vi "UHR-Fleezers Control (host) - Avogadro v2.vi"() -> ()   [LabVIEW 2014] (continued)
          frame Disabled {
            w2902 = FALSE ("Stop Flow")
            n1843 = local write "Stop Flow"(w2902) -> ()
            n1844 = local write "Sample Channel\nFlow"(w2902) -> ()
            n1845 = Concatenate Strings("stop" ("string"), "\r") -> (w2905:string)
            n1846 = VISA Write(VISA resource name=w2903, write buffer=w2905) -> ()  [unwired: 1 in, 3 out]
          }
          frame Enabled {
          }
        }
      }
      event "Flow rate (uL/h)": Value Change {
        n1847 = event-data() -> ()  [unwired: 7 out]
        n1848 = disable-structure shown="Disabled" {
          disable-tunnel: w2907 -> [w2909 _]
          frame Disabled {
            n1849 = Number To Decimal String(number="Flow rate (uL/h)") -> (decimal integer string=w2913:string)  [unwired: 1 in]
            n1850 = Concatenate Strings("irate  " ("string"), w2913, " u/h" ("string"), "\r") -> (w2912:string)
            n1851 = VISA Write(VISA resource name=w2909, write buffer=w2912) -> ()  [unwired: 1 in, 3 out]
          }
          frame Enabled {
          }
        }
      }
      event "Flush Sample": Value Change {
        n1852 = event-data() -> ()  [unwired: 7 out]
        n1853 = disable-structure shown="Disabled" {
          disable-tunnel: ["Flush Sample" _] -> w2916
          disable-tunnel: w2915 -> [w2922 _]
          frame Disabled {
            n1854 = flat-sequence {
              tunnel: w2922 -> [w2963]
              tunnel: [w2943] -> w2926
              tunnel: [w2939] -> w2925
              tunnel: ["Volume (uL)"] -> w2921
              tunnel: ["Flush rate (uL/m)"] -> w2920
              tunnel: w2926 -> [w2967]
              tunnel: [w2967] -> w2924
              tunnel: w2925 -> [w2966]
              tunnel: w2924 -> [w2972]
              frame #0 {
                # "set paramaters (rate, volume) for flush, clear volume"
                n1855 = Number To Decimal String(number="Flush rate (uL/m)") -> (decimal integer string=w2959:string)  [unwired: 1 in]
                n1856 = Concatenate Strings("irate  " ("string"), w2959, " u/m" ("string"), "\r") -> (w2961:string)
                n1857 = VISA Write(VISA resource name=w2963, write buffer=w2961) -> (VISA resource name out=w2957:refnum<visa-resource-name>)  [unwired: 1 in, 2 out]
                n1858 = Reciprocal(x="Flush rate (uL/m)") -> (1/x=w2942:dbl)
                n1859 = Number To Decimal String(number="Volume (uL)") -> (decimal integer string=w2948:string)  [unwired: 1 in]
                n1860 = Multiply(x="Volume (uL)", y=w2942) -> (x*y=w2941:dbl)
                n1861 = Concatenate Strings("tvolume  " ("string"), w2948, " u" ("string"), "\r") -> (w2946:string)
                n1862 = Multiply(x=w2941, y=60000.0) -> (x*y=w2939:dbl)
                n1863 = VISA Write(VISA resource name=w2957, write buffer=w2946) -> (VISA resource name out=w2945:refnum<visa-resource-name>)  [unwired: 1 in, 2 out]
                n1864 = Concatenate Strings("cvolume" ("string"), "\r") -> (w2944:string)
                n1865 = VISA Write(VISA resource name=w2945, write buffer=w2944) -> (VISA resource name out=w2955:refnum<visa-resource-name>)  [unwired: 1 in, 2 out]
                n1866 = Concatenate Strings("irun" ("string"), "\r") -> (w2953:string)
                n1867 = VISA Write(VISA resource name=w2955, write buffer=w2953) -> (VISA resource name out=w2943:refnum<visa-resource-name>)  [unwired: 1 in, 2 out]
              }
              frame #1 {
                # "Have to wait until\nflow is done to reset\nrate"
                n1868 = Add(x=w2966, y=100.0) -> (x+y=w2965:dbl)
                n1869 = Wait (ms)(milliseconds to wait=w2965) -> ()  [unwired: 1 out]
              }
              frame #2 {
                # "reset flow rate to usual flow rate"
                n1870 = local read "Flow rate (uL/h)"() -> (w2978:dbl)
                n1871 = Number To Decimal String(number=w2978) -> (decimal integer string=w2976:string)  [unwired: 1 in]
                n1872 = Concatenate Strings("irate  " ("string"), w2976, " u/h" ("string"), "\r") -> (w2974:string)
                n1873 = VISA Write(VISA resource name=w2972, write buffer=w2974) -> (VISA resource name out=w2968:refnum<visa-resource-name>)  [unwired: 1 in, 2 out]
                n1874 = Concatenate Strings("cvolume" ("string"), "\r") -> (w2969:string)
                n1875 = VISA Write(VISA resource name=w2968, write buffer=w2969) -> ()  [unwired: 1 in, 3 out]
              }
            }
            n1876 = local read "Save Event Log?"() -> (w2918:bool)
            n1877 = local read "Saving..."() -> (w2917:bool)
            n1878 = And(x=w2918, y=w2917) -> (x .and. y?=w2919:bool)
            n1879 = case shown="True" w2919 {
              tunnel: w2921 -> [_ w2928]
              tunnel: w2920 -> [_ w2927]
              frame False {
              }
              frame True {
                n1880 = Number To Decimal String(number=w2928) -> (decimal integer string=w2932:string)  [unwired: 1 in]
                n1881 = Number To Decimal String(number=w2927) -> (decimal integer string=w2934:string)  [unwired: 1 in]
                n1882 = local read "log file ref"() -> (w2929:refnum<file>)
                n1883 = local read "Time (s)"() -> (w2930:dbl)
                n1884 = Concatenate Strings("pump 2 flushing ", w2932, " uL at ", w2934, " ul/min") -> (w2936:string)
                n1885 = call "write to event log.vi"("log file ref"=w2929, "time"=w2930, "input string"=w2936) -> ()  [unwired: 8 in]
              }
            }
          }
          frame Enabled {
          }
        }
      }
      event "Flush Pump 3": Value Change {
        n1886 = event-data() -> ()  [unwired: 7 out]
        n1887 = disable-structure shown="Disabled" {
          disable-tunnel: ["Flush Pump 3" _] -> w2980
          disable-tunnel: w2979 -> [w2986 _]
          frame Disabled {
            n1888 = flat-sequence {
              tunnel: w2986 -> [w3001]
              tunnel: ["Flush rate (uL/m) P3"] -> w2982
              tunnel: ["Volume (uL) P3"] -> w2981
              frame #0 {
                # "set paramaters (rate, volume) for flush, clear volume"
                n1889 = Number To Decimal String(number="Flush rate (uL/m) P3") -> (decimal integer string=w3021:string)  [unwired: 1 in]
                n1890 = local write "Inject Pump 3"(TRUE ("Inject Pump 3")) -> ()
                n1891 = Concatenate Strings("irate  " ("string"), w3021, " u/m" ("string"), "\r") -> (w3023:string)
                n1892 = VISA Write(VISA resource name=w3001, write buffer=w3023) -> (VISA resource name out=w3019:refnum<visa-resource-name>)  [unwired: 1 in, 2 out]
                n1893 = Reciprocal(x="Flush rate (uL/m) P3") -> (1/x=w3005:dbl)
                n1894 = Number To Decimal String(number="Volume (uL) P3") -> (decimal integer string=w3010:string)  [unwired: 1 in]
                n1895 = Multiply(x="Volume (uL) P3", y=w3005) -> (x*y=w3004:dbl)
                n1896 = Concatenate Strings("tvolume  " ("string"), w3010, " u" ("string"), "\r") -> (w3008:string)
                n1897 = Multiply(x=w3004, y=60.0) -> (x*y=→"HP3 Flush Time (s)":dbl)
                n1898 = VISA Write(VISA resource name=w3019, write buffer=w3008) -> (VISA resource name out=w3007:refnum<visa-resource-name>)  [unwired: 1 in, 2 out]
                n1899 = Concatenate Strings("cvolume" ("string"), "\r") -> (w3006:string)
                n1900 = VISA Write(VISA resource name=w3007, write buffer=w3006) -> (VISA resource name out=w3017:refnum<visa-resource-name>)  [unwired: 1 in, 2 out]
                n1901 = Concatenate Strings("irun" ("string"), "\r") -> (w3015:string)
                n1902 = VISA Write(VISA resource name=w3017, write buffer=w3015) -> ()  [unwired: 1 in, 3 out]
              }
              frame #1 {
                "Flushing P3" <- TRUE ("Flushing P3")
              }
            }
            n1903 = local read "Save Event Log?"() -> (w2984:bool)
            n1904 = local read "Saving..."() -> (w2985:bool)
            n1905 = And(x=w2984, y=w2985) -> (x .and. y?=w2983:bool)
            n1906 = case shown="True" w2983 {
              tunnel: w2982 -> [_ w2989]
              tunnel: w2981 -> [_ w2988]
              frame False {
              }
              frame True {
                n1907 = Number To Decimal String(number=w2988) -> (decimal integer string=w2993:string)  [unwired: 1 in]
                n1908 = Number To Decimal String(number=w2989) -> (decimal integer string=w2995:string)  [unwired: 1 in]
                n1909 = local read "log file ref"() -> (w2990:refnum<file>)
                n1910 = local read "Time (s)"() -> (w2991:dbl)
                n1911 = Concatenate Strings("pump 3 flushing ", w2993, " uL at ", w2995, " ul/min") -> (w2997:string)
                n1912 = call "write to event log.vi"("log file ref"=w2990, "time"=w2991, "input string"=w2997) -> ()  [unwired: 8 in]
              }
            }
          }
          frame Enabled {
          }
        }
      }
      event "Flush Pump 1": Value Change {
        n1913 = event-data() -> ()  [unwired: 7 out]
        n1914 = disable-structure shown="Disabled" {
          disable-tunnel: ["Flush Pump 1" _] -> w3027
          disable-tunnel: w3026 -> [w3033 _]
          frame Disabled {
            n1915 = flat-sequence {
              tunnel: [w3054] -> w3035
              tunnel: w3033 -> [w3049]
              tunnel: ["Volume (uL) P1"] -> w3029
              tunnel: ["Flush rate (uL/m) P1"] -> w3028
              tunnel: w3035 -> [_]
              frame #0 {
                # "set paramaters (rate, volume) for flush, clear volume"
                n1916 = local write "Inject Pump 1"(TRUE ("Inject Pump 1")) -> ()
                n1917 = Number To Decimal String(number="Flush rate (uL/m) P1") -> (decimal integer string=w3070:string)  [unwired: 1 in]
                n1918 = Concatenate Strings("irate  " ("string"), w3070, " u/m" ("string"), "\r") -> (w3072:string)
                n1919 = VISA Write(VISA resource name=w3049, write buffer=w3072) -> (VISA resource name out=w3068:refnum<visa-resource-name>)  [unwired: 1 in, 2 out]
                n1920 = Reciprocal(x="Flush rate (uL/m) P1") -> (1/x=w3053:dbl)
                n1921 = Number To Decimal String(number="Volume (uL) P1") -> (decimal integer string=w3059:string)  [unwired: 1 in]
                n1922 = Multiply(x="Volume (uL) P1", y=w3053) -> (x*y=w3052:dbl)
                n1923 = Concatenate Strings("tvolume  " ("string"), w3059, " u" ("string"), "\r") -> (w3057:string)
                n1924 = Multiply(x=w3052, y=60.0) -> (x*y=→"HP1 Flush Time (s)":dbl)
                n1925 = VISA Write(VISA resource name=w3068, write buffer=w3057) -> (VISA resource name out=w3056:refnum<visa-resource-name>)  [unwired: 1 in, 2 out]
                n1926 = Concatenate Strings("cvolume" ("string"), "\r") -> (w3055:string)
                n1927 = VISA Write(VISA resource name=w3056, write buffer=w3055) -> (VISA resource name out=w3066:refnum<visa-resource-name>)  [unwired: 1 in, 2 out]
                n1928 = Concatenate Strings("irun" ("string"), "\r") -> (w3064:string)
                n1929 = VISA Write(VISA resource name=w3066, write buffer=w3064) -> (VISA resource name out=w3054:refnum<visa-resource-name>)  [unwired: 1 in, 2 out]
              }
              frame #1 {
                "Flushing P1" <- TRUE ("Flushing P3")
              }
            }
            n1930 = local read "Saving..."() -> (w3030:bool)
            n1931 = local read "Save Event Log?"() -> (w3031:bool)
            n1932 = And(x=w3031, y=w3030) -> (x .and. y?=w3032:bool)
            n1933 = case shown="True" w3032 {
              tunnel: w3029 -> [_ w3038]
              tunnel: w3028 -> [_ w3037]
              frame False {
              }
              frame True {
                n1934 = Number To Decimal String(number=w3038) -> (decimal integer string=w3042:string)  [unwired: 1 in]
                n1935 = Number To Decimal String(number=w3037) -> (decimal integer string=w3040:string)  [unwired: 1 in]
                n1936 = local read "log file ref"() -> (w3044:refnum<file>)
                n1937 = local read "Time (s)"() -> (w3045:dbl)
                n1938 = Concatenate Strings("pump 1 flushing ", w3042, " uL at ", w3040, " ul/min") -> (w3036:string)
                n1939 = call "write to event log.vi"("log file ref"=w3044, "time"=w3045, "input string"=w3036) -> ()  [unwired: 8 in]
              }
            }
          }
          frame Enabled {
          }
        }
      }
      event "Clear Volume": Value Change {
        n1940 = event-data() -> ()  [unwired: 7 out]
        n1941 = disable-structure shown="Disabled" {
          disable-tunnel: ["Clear Volume" _] -> w3076
          disable-tunnel: w3075 -> [w3077 _]
          frame Disabled {
            n1942 = Concatenate Strings("cvolume" ("string"), "\r") -> (w3078:string)
            n1943 = VISA Write(VISA resource name=w3077, write buffer=w3078) -> ()  [unwired: 1 in, 3 out]
          }
          frame Enabled {
          }
        }
      }
      event "Clear Volume P3": Value Change {
        n1944 = event-data() -> ()  [unwired: 7 out]
        n1945 = disable-structure shown="Disabled" {
          disable-tunnel: w3082 -> [w3084 _]
          frame Disabled {
            n1946 = Concatenate Strings("cvolume" ("string"), "\r") -> (w3085:string)
            n1947 = VISA Write(VISA resource name=w3084, write buffer=w3085) -> ()  [unwired: 1 in, 3 out]
            n1948 = local write "Clear Volume P3"(FALSE ("Clear Volume P3")) -> ()
          }
          frame Enabled {
          }
        }
      }
      event "Clear Volume P1": Value Change {
        n1949 = event-data() -> ()  [unwired: 7 out]
        n1950 = disable-structure shown="Disabled" {
          disable-tunnel: w3088 -> [w3090 _]
          frame Disabled {
            n1951 = Concatenate Strings("cvolume" ("string"), "\r") -> (w3091:string)
            n1952 = local write "Clear Volume P1"(FALSE ("Clear Volume P1")) -> ()
            n1953 = VISA Write(VISA resource name=w3090, write buffer=w3091) -> ()  [unwired: 1 in, 3 out]
          }
          frame Enabled {
          }
        }
      }
      event "Display On P3": Value Change {
        n1954 = event-data() -> ()  [unwired: 7 out]
        n1955 = disable-structure shown="Disabled" {
          disable-tunnel: w3094 -> [w3095 _]
          frame Disabled {
            n1956 = Select(t="dim 100", s="Display On P3", f="dim 0") -> (s? t:f=w3098:string)
            n1957 = Concatenate Strings(w3098, "\r") -> (w3100:string)
            n1958 = VISA Write(VISA resource name=w3095, write buffer=w3100) -> ()  [unwired: 1 in, 3 out]
          }
          frame Enabled {
          }
        }
      }
      event "Display On P1": Value Change {
        n1959 = event-data() -> ()  [unwired: 7 out]
        n1960 = disable-structure shown="Disabled" {
          disable-tunnel: w3102 -> [w3103 _]
          frame Disabled {
            n1961 = Select(t="dim 100", s="Display On P1", f="dim 0") -> (s? t:f=w3106:string)
            n1962 = Concatenate Strings(w3106, "\r") -> (w3108:string)
            n1963 = VISA Write(VISA resource name=w3103, write buffer=w3108) -> ()  [unwired: 1 in, 3 out]
          }
          frame Enabled {
          }
        }
      }
      event "Retract Pump 3": Value Change {
        n1964 = event-data() -> ()  [unwired: 7 out]
        n1965 = disable-structure shown="Disabled" {
          disable-tunnel: w3110 -> [w3111 _]
          frame Disabled {
            n1966 = local write "Retract Pump 3"(FALSE ("Retract Pump 3")) -> ()
            n1967 = case shown="True" "Retract Pump 3" {
              tunnel: w3111 -> [_ w3114]
              frame False {
              }
              frame True {
                n1968 = Number To Decimal String(number="Retract Rate (uL/m)") -> (decimal integer string=w3132:string)  [unwired: 1 in]
                n1969 = Concatenate Strings("wrate  " ("string"), w3132, " u/m" ("string"), "\r") -> (w3134:string)
                n1970 = VISA Write(VISA resource name=w3114, write buffer=w3134) -> (VISA resource name out=w3125:refnum<visa-resource-name>)  [unwired: 1 in, 2 out]
                n1971 = Number To Decimal String(number="Retract Vol 3 (uL)") -> (decimal integer string=w3127:string)  [unwired: 1 in]
                n1972 = Concatenate Strings("tvolume  " ("string"), w3127, " u" ("string"), "\r") -> (w3124:string)
                n1973 = VISA Write(VISA resource name=w3125, write buffer=w3124) -> (VISA resource name out=w3120:refnum<visa-resource-name>)  [unwired: 1 in, 2 out]
                n1974 = Concatenate Strings("cvolume" ("string"), "\r") -> (w3121:string)
                n1975 = VISA Write(VISA resource name=w3120, write buffer=w3121) -> (VISA resource name out=w3115:refnum<visa-resource-name>)  [unwired: 1 in, 2 out]
                n1976 = Concatenate Strings("wrun" ("string"), "\r") -> (w3116:string)
                n1977 = VISA Write(VISA resource name=w3115, write buffer=w3116) -> ()  [unwired: 1 in, 3 out]
              }
            }
          }
          frame Enabled {
          }
        }
      }
      event "Retract Pump 1": Value Change {
        n1978 = event-data() -> ()  [unwired: 7 out]
        n1979 = disable-structure shown="Disabled" {
          disable-tunnel: w3136 -> [w3137 _]
          frame Disabled {
            n1980 = local write "Retract Pump 1"(FALSE ("Retract Pump 1")) -> ()
            n1981 = case shown="True" "Retract Pump 1" {
              tunnel: w3137 -> [_ w3142]
              frame False {
              }
              frame True {
                n1982 = local read "Retract Rate (uL/m)"() -> (w3140:dbl)
                n1983 = Number To Decimal String(number=w3140) -> (decimal integer string=w3158:string)  [unwired: 1 in]
                n1984 = Concatenate Strings("wrate  " ("string"), w3158, " u/m" ("string"), "\r") -> (w3160:string)
                n1985 = VISA Write(VISA resource name=w3142, write buffer=w3160) -> (VISA resource name out=w3152:refnum<visa-resource-name>)  [unwired: 1 in, 2 out]
                n1986 = Number To Decimal String(number="Retract Vol 1 (uL)") -> (decimal integer string=w3154:string)  [unwired: 1 in]
                n1987 = Concatenate Strings("tvolume  " ("string"), w3154, " u" ("string"), "\r") -> (w3151:string)
                n1988 = VISA Write(VISA resource name=w3152, write buffer=w3151) -> (VISA resource name out=w3148:refnum<visa-resource-name>)  [unwired: 1 in, 2 out]
                n1989 = Concatenate Strings("cvolume" ("string"), "\r") -> (w3149:string)
                n1990 = VISA Write(VISA resource name=w3148, write buffer=w3149) -> (VISA resource name out=w3143:refnum<visa-resource-name>)  [unwired: 1 in, 2 out]
                n1991 = Concatenate Strings("wrun" ("string"), "\r") -> (w3144:string)
                n1992 = VISA Write(VISA resource name=w3143, write buffer=w3144) -> ()  [unwired: 1 in, 3 out]
              }
            }
          }
          frame Enabled {
          }
        }
      }
      event "Flip Green Filter": Value Change {
        n1993 = event-data() -> ()  [unwired: 7 out]
        n1994 = Not(x="Flip Green Filter") -> (.not. x?=w3163:bool)
        n1995 = local write "Flip Green Filter"(w3163) -> ()
        n1996 = flat-sequence {
          tunnel: [w3172] -> w3168
          tunnel: [w3171] -> w3167
          tunnel: w3162 -> [w3170]
          tunnel: [w3175] -> w3166
          tunnel: w3168 -> [w3175]
          tunnel: [w3174] -> w3165
          tunnel: w3167 -> [w3174]
          tunnel: w3166 -> [w3179]
          tunnel: w3165 -> [w3178]
          tunnel: [w3177] -> w3169
          frame #0 {
            n1997 = xnode "Read/Write Control"("FPGA VI Reference In"=w3170, "Green Filter Flipper"=TRUE) -> ("FPGA VI Reference Out"=w3172:T40, "error out"=w3171:errorcluster)  [unwired: 1 in]
          }
          frame #1 {
            n1998 = Wait (ms)(milliseconds to wait=u32 100) -> ()  [unwired: 1 out]
          }
          frame #2 {
            n1999 = xnode "Read/Write Control"("FPGA VI Reference In"=w3179, "error in"=w3178, "Green Filter Flipper"=FALSE) -> ("error out"=w3177:errorcluster)  [unwired: 1 out]
          }
        }
      }
      event "Pump 1 contents", "Pump 3 contents": Value Change {
        n2000 = event-data() -> ()  [unwired: 7 out]
        n2001 = local read "Pump 1 contents"() -> (→"Pump 1 cont disp":string)
        n2002 = local read "Pump 3 contents"() -> (→"Pump 3 cont disp":string)
      }
      event "Reset Trap Pos. FB": Value Change {
        n2003 = event-data() -> ()  [unwired: 7 out]
        n2004 = xnode "Read/Write Control"("FPGA VI Reference In"=w3183, "Trap Pos. FB Reset"="Reset Trap Pos. FB") -> ()  [unwired: 1 in, 2 out]
      }
      event "Rem fb disp offset": Value Change {
        n2005 = event-data() -> ()  [unwired: 7 out]
        n2006 = local write "Rem fb disp offset"(FALSE ("Rem fb disp offset")) -> ()
        n2007 = local read "Mean Trap Positions (nm)"() -> (w3186:T6)
        n2008 = local read "FB Trap Pos Offset"() -> (w3188:dbl)
        n2009 = Unbundle By Name(w3186) -> ("T1 X"=w3185:dbl)
        n2010 = Subtract(x=w3188, y=w3185) -> (x-y=w3187:dbl)
        n2011 = local write "FB Trap Pos Offset"(w3187) -> ()
      }
      event "Threshold (nm)": Value Change {
        n2012 = event-data() -> ()  [unwired: 7 out]
        n2013 = flat-sequence {
          tunnel: [w3193] -> w3191
          tunnel: w3190 -> [w3192]
          tunnel: w3191 -> [w3204]
          frame #0 {
            n2014 = xnode "Read/Write Control"("FPGA VI Reference In"=w3192) -> ("FPGA VI Reference Out"=w3196:T40, "error out"=w3195:errorcluster, "FPGA TTrig Thresh"=w3197:i64)  [unwired: 1 in]
            n2015 = local read "Threshold stored (nm)"() -> (w3203:dbl)
            n2016 = local read "Threshold (nm)"() -> (w3193:dbl)
            n2017 = local read "AOM X Cal (nm/MHz)"() -> (w3201:dbl)
            n2018 = Subtract(x=w3193, y=w3203) -> (x-y=w3202:dbl)
            n2019 = Divide(x=w3202, y=w3201) -> (x/y=w3199:dbl)
            n2020 = call "IR AOM freq to word.vi"("Frequency In (MHz)"=w3199) -> ("Frequency Word Out (double)"=w3200:dbl)
            n2021 = To Quad Integer(1:w3200) -> (0:w3198:i64)
            n2022 = Add(x=w3197, y=w3198) -> (x+y=w3194:i64)
            n2023 = xnode "Read/Write Control"("FPGA VI Reference In"=w3196, "error in"=w3195, "FPGA TTrig Thresh"=w3194) -> ()  [unwired: 2 out]
          }
          frame #1 {
            "Threshold stored (nm)" <- w3204
          }
        }
      }
      event "FB Trig Integrate": Value Change {
        n2024 = event-data() -> ()  [unwired: 7 out]
        n2025 = local read "FB Trig Integrate"() -> (w3207:u32)
        n2026 = xnode "Read/Write Control"("FPGA VI Reference In"=w3205, "FB Trig Integrate"=w3207) -> ("error out"=w3206:errorcluster)  [unwired: 1 in, 1 out]
      }
      event "11": Value Change {
        n2027 = event-data() -> ()  [unwired: 7 out]
        n2028 = local read "11"() -> (w3208:bool)
        n2029 = case shown="True" w3208 {
          frame False {
          }
          frame True {
            n2030 = local read "Messages"() -> (w3210:string)
            n2031 = call "Update messages.vi"("Message to add"="You kicked it up to 11!", "Old message string"=w3210) -> ("New message string"=w3211:string)
            n2032 = call <vilib>:"Beep.vi"() -> ()  [unwired: 12 in]
            n2033 = local write "Messages"(w3211) -> ()
          }
        }
      }
      event "Trap Pos. FB ON": Value Change {
        w3218 = 6.0  # clock mult.
        w3217 = 49152000.0  # TCXO frequ.
        n2034 = event-data() -> ()  [unwired: 7 out]
        n2035 = xnode "Read/Write Control"("FPGA VI Reference In"=w3212) -> ("FPGA VI Reference Out"=w3214:T40, "BD1 Frequency Out 1"=w3215:u64)  [unwired: 1 in, 1 out]
        n2036 = To Double Precision Float(number=w3215) -> (double precision float=w3219:dbl)
        n2037 = Multiply(x=w3217, y=w3218) -> (x*y=w3220:dbl)
        n2038 = Multiply(x=w3219, y=w3220) -> (x*y=w3221:dbl)
        n2039 = Scale By Power Of 2(n=-48, x=w3221) -> (x*2^n=w3223:dbl)
        n2040 = Divide(x=w3223, y=1000000.0) -> (x/y=w3216:dbl)
        n2041 = flat-sequence {
          tunnel: w3214 -> [w3229]
          tunnel: [w3228] -> w3225
          tunnel: "Trap Pos. FB ON" -> [w3227]
          tunnel: w3215 -> [w3226]
          tunnel: w3225 -> [w3235]
          tunnel: "Trap Pos. FB ON" -> [w3234]
          tunnel: w3216 -> [w3237]
          tunnel: "Trap Pos. FB ON" -> [w3236]
          frame #0 {
            n2042 = case shown="False" w3227 {
              tunnel: w3229 -> [w3231 w3233]
              tunnel: [w3232 w3233] -> w3228
              tunnel: w3226 -> [w3230 _]
              frame False {
                n2043 = xnode "Read/Write Control"("FPGA VI Reference In"=w3231, "BD 1 Frequency 1"=w3230) -> ("FPGA VI Reference Out"=w3232:T40)  [unwired: 1 in, 1 out]
              }
              frame True {
              }
            }
          }
          frame #1 {
            n2044 = xnode "Read/Write Control"("FPGA VI Reference In"=w3235, "Force feedback"=w3234) -> ()  [unwired: 1 in, 2 out]
          }
          frame #2 {
            n2045 = case shown="False" w3236 {
              tunnel: w3237 -> [w3238 _]
              frame False {
                n2046 = property on="BD 1 Frequency 1 (MHz)" class="DigNum (strict)"("Val(Sgnl)"=w3238) -> ()  [unwired: 2 in, 2 out]
              }
              frame True {
              }
            }
          }
        }
      }
      event "Remove Action Offset": Value Change {
        n2047 = event-data() -> ()  [unwired: 7 out]
        n2048 = local write "Remove Action Offset"(FALSE ("Remove Action Offset")) -> ()
        n2049 = local read "Trap Pos. FB Mult Factor"() -> (w3244:i64)
        n2050 = local read "Trap Pos FB Action"() -> (w3242:i64)
        n2051 = local read "Trap Pos. FB Offset Factor"() -> (w3240:i64)
        n2052 = Multiply(x=w3244, y=w3242) -> (x*y=w3243:i64)
        n2053 = Add(x=w3243, y=w3240) -> (x+y=w3241:i64)
        n2054 = local write "Trap Pos. FB Offset Factor"(w3241) -> ()
        n2055 = xnode "Read/Write Control"("FPGA VI Reference In"=w3239, "Trap Pos. FB Offset Factor"=w3241) -> ()  [unwired: 1 in, 2 out]
      }
      event "Remove Unwinding Offset": Value Change {
        n2056 = event-data() -> ()  [unwired: 7 out]
        n2057 = local write "Remove Unwinding Offset"(FALSE ("Remove Action Offset")) -> ()
        n2058 = local read "Trap Pos. FB Mult Factor"() -> (w3258:i64)
        n2059 = local read "Trap Pos FB Action"() -> (w3256:i64)
        n2060 = local read "Trap Pos. FB Offset Factor"() -> (w3255:i64)
        n2061 = Multiply(x=w3258, y=w3256) -> (x*y=w3257:i64)
        n2062 = local read "Trap Pos. FB Mult Factor"() -> (w3254:i64)
        n2063 = Add(x=w3257, y=w3255) -> (x+y=w3248:i64)
        n2064 = Multiply(x=32768, y="factor") -> (x*y=w3251:dbl)
        n2065 = Multiply(x=w3251, y=w3254) -> (x*y=w3253:dbl)
        n2066 = Subtract(x=w3248, y=w3253) -> (x-y=w3252:dbl)
        n2067 = To Quad Integer(1:w3252) -> (0:w3247:i64)
        n2068 = xnode "Read/Write Control"("FPGA VI Reference In"=w3246, "Trap Pos. FB Offset Factor"=w3247) -> ()  [unwired: 1 in, 2 out]
        n2069 = local write "Trap Pos. FB Offset Factor"(w3247) -> ()
      }
      event "Trap Pos. FB Range", "Trap Pos. FB Gains", "Trap Pos. FB Mult Factor", "Trap Pos. FB Offset Factor", "Trap Pos FB Negate Action", "Trap Pos FB Monitor\nT1 or T2", "Differential FB?", "Negate Diff?": Value Change {
        n2070 = event-data() -> ()  [unwired: 7 out]
        n2071 = local read "Negate Diff?"() -> (w3263:bool)
        n2072 = xnode "Read/Write Control"("FPGA VI Reference In"=w3262, "Trap Pos. FB Gains"="Trap Pos. FB Gains", "Trap pos. FB Range"="Trap Pos. FB Range", "Trap Pos. FB Mult Factor"="Trap Pos. FB Mult Factor", "Trap Pos. FB Offset Factor"="Trap Pos. FB Offset Factor", "Trap Pos FB Negate Action"="Trap Pos FB Negate Action", "Trap Pos FB Monitor T1 or T2"="Trap Pos FB Monitor\nT1 or T2", "AI1 X Scale"="Trap Pos. AI1 X Pre-scale", "Negate Diff?"=w3263, "Diff FB Measurement?"="Differential FB?") -> ()  [unwired: 1 in, 2 out]
      }
      event "Trap Pos FB SP", "Trap Pos FB SP 2", "Use SP 2": Value Change {
        n2073 = event-data() -> ()  [unwired: 7 out]
        n2074 = Select(t="Trap Pos FB SP 2", s="Use SP 2", f="Trap Pos FB SP") -> (s? t:f=w3271:fxp<+/-,16,1>)
        n2075 = xnode "Read/Write Control"("FPGA VI Reference In"=w3270, "Trap Pos. FB SP"=w3271) -> ()  [unwired: 1 in, 2 out]
      }
      event "Offset SP2 from SP1": Value Change {
        n2076 = event-data() -> ()  [unwired: 7 out]
        n2077 = local read "Trap Pos FB SP"() -> (w3277:fxp<+/-,16,1>)
        n2078 = Add(x=w3277, y="SP2 Offset") -> (x+y=w3275:fxp<+/-,16,1>)
        n2079 = property on="Trap Pos FB SP 2" class="DigNum (strict)"("Val(Sgnl)"=w3275) -> ()  [unwired: 2 in, 2 out]
        n2080 = local write "Offset SP2 from SP1"(FALSE ("Offset SP2 from SP1")) -> ()
      }
      event "Set Reading to\nSetpoint": Value Change {
        # "This is the actual PID input signal"
        n2081 = event-data() -> ()  [unwired: 7 out]
        n2082 = local write "Set Reading to\nSetpoint"(FALSE ("Set SP to Reading")) -> ()
        n2083 = xnode "Read/Write Control"("FPGA VI Reference In"=w3281) -> ("FPGA VI Reference Out"=w3284:T40, "error out"=w3283:errorcluster, "Trap Pos FB Int-Norm Signal"=w3282:fxp<+/-,16,1>, "BD1 Frequency Out 1"=w3280:u64)  [unwired: 1 in]
        n2084 = local read "Differential FB?"() -> (w3285:bool)
        n2085 = case shown="False" w3285 {
          tunnel: [w3314 w3321] -> w3279
          tunnel: w3282 -> [w3312 w3321]
          frame False {
            n2086 = local read "Trap Pos FB Monitor\nT1 or T2"() -> (w3317:bool)
            n2087 = local read "Trap X AI1 (DMA)"() -> (w3320:T23)
            n2088 = Unbundle By Name(w3320) -> ("Set 1"=w3319:fxp<+/-,16,1>, "Set 2"=w3318:fxp<+/-,16,1>)
            n2089 = Select(t=w3319, s=w3317, f=w3318) -> (s? t:f=w3316:fxp<+/-,16,1>)
            n2090 = Not(x="Set SP Using...") -> (.not. x?=w3313:bool)
            n2091 = Select(t=w3312, s=w3313, f=w3316) -> (s? t:f=w3314:fxp<+/-,16,1>)
          }
          frame True {
          }
        }
        n2092 = disable-structure shown="Disabled" {
          disable-tunnel: _ -> [w3290 _]
          disable-tunnel: w3280 -> [w3289 _]
          disable-tunnel: w3279 -> [w3288 _]
          frame Disabled {
            n2093 = case shown="True" w3290 {
              tunnel: [w3291 w3293] -> w3287
              tunnel: w3288 -> [w3291 w3292]
              tunnel: w3289 -> [_ w3311]
              frame False {
              }
              frame True {
                w3309 = 6.0  # clock mult.
                w3310 = 49152000.0  # TCXO frequ.
                # "Added by Ronen - for the real time\nchange of the setpoint to accomodate \nchanges in the offset."
                n2094 = To Double Precision Float(number=w3311) -> (double precision float=w3308:dbl)
                n2095 = local read "BD 1 Frequency 2 (MHz)"() -> (w3301:dbl)
                n2096 = Multiply(x=w3310, y=w3309) -> (x*y=w3307:dbl)
                n2097 = Multiply(x=w3308, y=w3307) -> (x*y=w3306:dbl)
                n2098 = local read "Offset file step size"() -> (w3299:dbl)
                n2099 = Scale By Power Of 2(n=-48, x=w3306) -> (x*2^n=w3304:dbl)
                n2100 = Divide(x=w3304, y=1000000.0) -> (x/y=w3302:dbl)
                n2101 = Subtract(x=w3301, y=w3302) -> (x-y=w3300:dbl)
                n2102 = Divide(x=w3300, y=w3299) -> (x/y=w3298:dbl)
                n2103 = local read item#-1() -> (w3296)
                n2104 = To Long Integer(number=w3298) -> (32bit integer=w3297:i32)
                n2105 = Index Array(array=w3296, index=w3297) -> (element=w3295)
                n2106 = To Fixed-Point(number=w3295) -> (fixed-point=w3294:fxp<+/-,16,1>)  [unwired: 1 in]
                n2107 = Add(x=w3292, y=w3294) -> (x+y=w3293:fxp<+/-,17,2>)
              }
            }
            "Offset corrected setpoint" <- w3287
          }
          frame Enabled {
          }
        }
        n2108 = local write "Trap Pos FB SP"(w3279) -> ()
        n2109 = xnode "Read/Write Control"("FPGA VI Reference In"=w3284, "error in"=w3283, "Trap Pos. FB SP"=w3279) -> ()  [unwired: 2 out]
      }
      event "Trap Pos. FB Out Scale 2^n": Value Change {
        n2110 = event-data() -> ()  [unwired: 7 out]
        n2111 = Scale By Power Of 2(n="Trap Pos. FB Out Scale 2^n", x=ext 1.0) -> (x*2^n=w3322:ext)
        n2112 = property on="Trap Pos. FB Mult Factor" class="DigNum (strict)"("Val(Sgnl)"=w3322) -> ()  [unwired: 2 in, 2 out]
      }
      event "Trap Pos FB Int Count": Value Change {
        n2113 = event-data() -> ()  [unwired: 7 out]
        n2114 = xnode "Read/Write Control"("FPGA VI Reference In"=w3325, "Trap Pos FB Int Count"="Trap Pos FB Int Count") -> ()  [unwired: 1 in, 2 out]
      }
      event "Display Saved Data": Value Change {
        n2115 = event-data() -> ()  [unwired: 7 out]
        n2116 = case shown="\"Amp Current\"" "Display Saved Data" {
          frame "Bead Seperation", Default {
            n2117 = property on="Amp current" class="WFGraph (strict)"("Visible"=FALSE) -> ()  [unwired: 2 in, 2 out]
            n2118 = property on="Trap Delta Graph" class="WFGraph (strict)"("Visible"=TRUE) -> ()  [unwired: 2 in, 2 out]
            n2119 = property on="Saved trap pos" class="WFGraph (strict)"("Visible"=FALSE) -> ()  [unwired: 2 in, 2 out]
          }
          frame "Amp Current" {
            n2120 = property on="Saved trap pos" class="WFGraph (strict)"("Visible"=FALSE) -> ()  [unwired: 2 in, 2 out]
            n2121 = property on="Trap Delta Graph" class="WFGraph (strict)"("Visible"=FALSE) -> ()  [unwired: 2 in, 2 out]
            n2122 = property on="Amp current" class="WFGraph (strict)"("Visible"=TRUE) -> ()  [unwired: 2 in, 2 out]
          }
          frame "Trap Position" {
            n2123 = property on="Saved trap pos" class="WFGraph (strict)"("Visible"=TRUE) -> ()  [unwired: 2 in, 2 out]
            n2124 = property on="Trap Delta Graph" class="WFGraph (strict)"("Visible"=FALSE) -> ()  [unwired: 2 in, 2 out]
            n2125 = property on="Amp current" class="WFGraph (strict)"("Visible"=FALSE) -> ()  [unwired: 2 in, 2 out]
          }
        }
      }
      event "Calibration": Value Change {
        n2126 = event-data() -> ()  [unwired: 7 out]
        n2127 = local read "Calibration"() -> (w3351:u16)
        n2128 = Select(t="X" ("Label.Text"), s=TRUE, f="Y" ("Label.Text")) -> (s? t:f=w3348:string)
        n2129 = case shown="2" w3351 {
          tunnel: ["Position (V)" ("Label.Text") "Position (nm)" ("Label.Text") "Force (pN)" ("Label.Text")] -> w3345
          tunnel: [" (V)" ("Label.Text") " (nm)" ("Label.Text") " (pN)" ("Label.Text")] -> w3342
          frame 0, Default {
          }
          frame 1 {
          }
          frame 2 {
          }
        }
        n2130 = Concatenate Strings("T1 " ("Label.Text"), w3348) -> (w3344:string)
        n2131 = Concatenate Strings("T2 " ("Label.Text"), w3348) -> (w3343:string)
        n2132 = property on="Force" class="WFChart (strict)"("YScale.NameLbl.Text"=w3345) -> ()  [unwired: 2 in, 2 out]
        n2133 = Concatenate Strings("Mean" ("Label.Text"), w3342) -> (w3341:string)
        n2134 = Concatenate Strings(w3344, w3342) -> (w3340:string)
        n2135 = Concatenate Strings(w3343, w3342) -> (w3339:string)
        n2136 = Concatenate Strings("Difference" ("Label.Text"), w3342) -> (w3338:string)
        n2137 = property on="Mean" class="DigNum (strict)"("Caption.Text"=w3341) -> ()  [unwired: 2 in, 2 out]
        n2138 = property on="T1 X" class="DigNum (strict)"("Caption.Text"=w3340) -> ()  [unwired: 2 in, 2 out]
        n2139 = property on="T2 X" class="DigNum (strict)"("Caption.Text"=w3339) -> ()  [unwired: 2 in, 2 out]
        n2140 = property on="Difference" class="DigNum (strict)"("Caption.Text"=w3338) -> ()  [unwired: 2 in, 2 out]
      }
      event "Base N trap periods", "Period scale factor", "Trap osc amp (MHz)", "Cal sets to save", "# Samples/trap", "Total Counts (ticks)": Value Change {
        w3360 = 1.0
        w3366 = u32 0 ("y")
        # "scales 0 to 2pi"
        # "Create vector of trap offset (oscillation) values."
        # "Compute oscillation period as a multiple of the trap period. Should also fit nicely as a factor of the DMA period.\nCompare ticks for accurate commensurability check."
        # "Oscillation frequency needs to be commensurate\nwith the data save time."
        # "Be commensurate with total save time/100 (or so). That way you are guaranteed you can average spectra at least 100x."
        n2141 = event-data() -> ()  [unwired: 7 out]
        n2142 = local read "Total Counts (ticks)"() -> (w3382:u16)
        n2143 = To Unsigned Long Integer(number=w3382) -> (unsigned 32bit integer=w3392:u32)
        n2144 = Multiply "Base osc period (ticks)"(x=w3392, y="Base N trap periods") -> (x*y=w3383:u32)
        n2145 = local read "# Samples/trap"() -> (w3387:u32)
        n2146 = Multiply "Scaled osc period (ticks)"(x=w3383, y="Period scale factor") -> (x*y=w3384:dbl)
        n2147 = Multiply(x="Base N trap periods", y="Period scale factor") -> ()  [unwired: 1 out]
        n2148 = local read "Cal sets to save"() -> (w3388:u32)
        n2149 = To Unsigned Quad Integer(1:w3384) -> (0:w3374:u64)
        n2150 = for "vector 0 to N -1" {
          N: w3360 -> [_]
          tunnel: [w3409] -> w3380 mode=indexing
          i -> [w3409]
        }
        n2151 = Multiply "Ticks/DMA"(x=w3387, y=w3392) -> (x*y=w3391:u32)
        n2152 = Multiply "Scaled osc period (s)"(x=w3374, y=2.5e-08) -> (x*y=w3386:dbl)
        "Trap OSC Period (s)" <- w3386
        n2153 = Reciprocal(x=w3386) -> (1/x=→"A cal freq (Hz)":dbl)
        n2154 = Multiply(x=w3380, y=6.283185307179586) -> (x*y=w3395:dbl[])
        n2155 = Quotient & Remainder(x=w3391, y=w3374) -> (x-y*floor(x/y)=w3367:u64, floor(x/y)=→"N osc / DMA":u64)
        "DMA remainder" <- w3367
        n2156 = Multiply "Total trap ticks"(x=w3388, y=w3391) -> (x*y=w3375:u32)
        n2157 = Divide(x=w3395, y=w3360) -> (x/y=w3396:dbl[])
        n2158 = Sine(x=w3396) -> (sin(x)=w3397:dbl[])
        n2159 = Quotient & Remainder(x=w3375, y=100) -> (x-y*floor(x/y)=w3370:u32, floor(x/y)=w3390:u32)
        "Total save/100 remainder" <- w3370
        n2160 = Multiply "Single period osc vector"(x=w3397, y="Trap osc amp (MHz)") -> (x*y=w3373:dbl[])
        n2161 = Quotient & Remainder(x=w3390, y=w3374) -> (x-y*floor(x/y)=w3369:u64, floor(x/y)=→"N osc/ (total save/100)":u64)
        "(total save/100) /osc period remainder" <- w3369
        n2162 = Quotient & Remainder(x=w3375, y=w3374) -> (x-y*floor(x/y)=w3368:u64)  [unwired: 1 out]
        "N trap osc periods per save remainder" <- w3368
        n2163 = call "IR AOM freq to word - vec.vi"("Frequency In (double vec, MHz)"=w3373) -> ("Frequency Word Out"=w3372:dbl[])
        n2164 = To Quad Integer(1:w3372) -> (0:w3371:i64[])
        n2165 = disable-structure shown="Disabled" {
          disable-tunnel: w3379 -> [w3401 _]
          disable-tunnel: w3371 -> [w3399 _]
          frame Disabled {
            n2166 = xnode "Read/Write Control"("FPGA VI Reference In"=w3401) -> ("FPGA VI Reference Out"=w3400:T40)  [unwired: 3 in, 1 out]
            n2167 = flat-sequence {
              tunnel: w3399 -> [w3404]
              tunnel: w3400 -> [w3403]
              frame #0 {
                n2168 = for "Write data to fpga memory" {
                  tunnel: w3403 -> [w3406]
                  tunnel: w3404 -> [_] mode=indexing
                  (unwired) TRUE ("Ready Write")
                  n2169 = xnode "Read/Write Control"("FPGA VI Reference In"=w3406) -> ("FPGA VI Reference Out"=w3405:T40)  [unwired: 4 in, 1 out]
                  n2170 = while {
                    tunnel: w3405 -> [w3407]
                    stop <- _ continue-if-true
                    n2171 = xnode "Read/Write Control"("FPGA VI Reference In"=w3407) -> ()  [unwired: 1 in, 3 out]
                  }
                }
                "Writing waveform to fpga memory" <- TRUE ("Writing waveform to fpga memory")
              }
              frame #1 {
                n2172 = local write "Writing waveform to fpga memory"(FALSE ("Writing waveform to fpga memory")) -> ()
              }
            }
          }
          frame Enabled {
          }
        }
        n2173 = Equal?(x=w3369, y=w3366) -> (x = y?=w3364:bool)
        n2174 = Equal?(x=w3370, y=w3366) -> (x = y?=w3365:bool)
        n2175 = Equal?(x=w3367, y=w3366) -> (x = y?=w3362:bool)
        n2176 = Equal?(x=w3368, y=w3366) -> (x = y?=w3363:bool)
        n2177 = Compound Arithmetic op=AND(w3365, w3364, w3363, w3362) -> (→"Good freq?":bool)
      }
      event "Osc trap cont.", "Osc traps", "T1 Osc Enable", "T2 Osc Enable": Value Change {
        n2178 = event-data() -> ()  [unwired: 7 out]
        n2179 = disable-structure shown="Disabled" {
          disable-tunnel: w3410 -> [w3413 _]
          frame Disabled {
            n2180 = xnode "Read/Write Control"("FPGA VI Reference In"=w3413, "Trap 1 osc enable"="T1 Osc Enable", "Trap 2 osc enable"="T2 Osc Enable") -> ()  [unwired: 1 in, 2 out]
          }
          frame Enabled {
          }
        }
      }
      event "Pressure Pump Voltage (+/-10V)": Value Change {
        n2181 = event-data() -> ()  [unwired: 7 out]
        n2182 = disable-structure shown="Disabled" {
          disable-tunnel: w3414 -> [w3418 _]
          frame Disabled {
            n2183 = Divide(x="Pressure Pump Voltage (+/-10V)", y=10.0) -> (x/y=w3415:dbl)
            n2184 = Multiply(x=w3415, y=32767.0) -> (x*y=w3416:dbl)
            n2185 = xnode "Read/Write Control"("FPGA VI Reference In"=w3418, "Pressure Pump"=w3416) -> ()  [unwired: 1 in, 2 out]
          }
          frame Enabled {
          }
        }
      }
      event "Dynamic Force FB (ronen)": Value Change {
        # "Added by ronen - for feedback on trap position by changing the actual frequency and not the set frequency - for increasing the range of feedback."
        n2186 = event-data() -> ()  [unwired: 7 out]
        n2187 = xnode "Read/Write Control"("FPGA VI Reference In"=w3422, "Dynamic Force FB (Ronen)"="Dynamic Force FB (ronen)") -> ()  [unwired: 1 in, 2 out]
      }
      event "Read Setpoint Correction File": Value Change {
        n2188 = event-data() -> ()  [unwired: 7 out]
        n2189 = Open/Create/Replace File(file path (use dialog)="Setpoint Correction Offset File", operation (0:open)=T52."open", access (0:read/write)=enum16{"read/write", "read-only", "write-only"}."read-only") -> (refnum out=w3433:refnum<file>)  [unwired: 1 in, 4 out]
        n2190 = local write "Read Setpoint Correction File"(FALSE ("Read Setpoint Correction File")) -> ()
        n2191 = Deny Access(7:w3433) -> (3:w3432:refnum<file>)  [unwired: 1 in, 2 out]
        n2192 = Read from Binary File(5:0.0, 9:T53."big-endian, network order" ("byte order (0:big-endian, network order)"), 10:-1 ("count (1)"), 11:w3432) -> (2:w3423:dbl[], 3:w3431:refnum<file>)  [unwired: 1 in, 3 out]
        n2193 = Close File(refnum=w3431) -> ()  [unwired: 1 in, 2 out]
        n2194 = local read "Multiple-MCL offset?"() -> (w3425:bool)
        n2195 = local write "Raw offsets"(w3423) -> ()
        n2196 = case shown="True" w3425 {
          tunnel: w3423 -> [w3444 w3451]
          tunnel: [w3443 w3449] -> w3428
          tunnel: [w3442 w3448] -> w3427
          frame False {
            # "If not doing multiple offset, same calculation as before"
            n2197 = Decimate 1D Array(w3444) -> (w3443:dbl[], w3442:dbl[])
            n2198 = local read "Two Trap Offset Values"() -> (w3441:T31)
            n2199 = Bundle By Name(cluster=w3441, "Trap 1X offset"=w3443, "Trap 2X offset"=w3442) -> (w3440:T31)
            n2200 = local write "Two Trap Offset Values"(w3440) -> ()
          }
          frame True {
            w3446 = 0.0
            # "When doing multiple offset: separate data to different scans, make array of clusters of 1x,1y,2x,2y,3x,3y arrays"
            n2201 = local read "MCL offset scanning range (V)"() -> (w3452:T4)
            n2202 = local read "Offset file step size"() -> (w3450:dbl)
            n2203 = Build Array(w3446, w3446, w3446, w3446, w3446, w3446) -> (w3445:dbl[])
            n2204 = call "generate multiple MCL offset.vi"("Offset array"=w3451, "offset file step size"=w3450, "MCL offset scanning range (V)"=w3452, "Corrections"=w3445) -> ("B_X mean out"=w3448:dbl[], "A_X mean out"=w3449:dbl[], "Output array"=w3447:T30)
            n2205 = local write "Multi-MCL offset array"(w3447) -> ()
          }
        }
        n2206 = local read "B factor"() -> (w3424:dbl)
        n2207 = Multiply(x=w3427, y=w3424) -> (x*y=w3429:dbl[])
        n2208 = Subtract(x=w3428, y=w3429) -> (x-y=w3426:dbl[])
        n2209 = property on="Setpoint offset\ncorrection values" class="Arr (strict)"("Val(Sgnl)"=w3426) -> ()  [unwired: 2 in, 2 out]
      }
      event "B factor", "Setpoint offset\ncorrection values", "Target Force (pN)": Value Change {
        w3483 = 6.0  # clock mult.
        w3484 = 49152000.0  # TCXO frequ.
        n2210 = event-data() -> ()  [unwired: 7 out]
        n2211 = local read "B factor"() -> (w3485:dbl)
        n2212 = xnode "Read/Write Control"("FPGA VI Reference In"=w3486, "B factor"=w3485) -> ("BD1 Frequency Out 1"=w3476:u64)  [unwired: 1 in, 2 out]
        n2213 = To Double Precision Float(number=w3476) -> (double precision float=w3482:dbl)
        n2214 = local read "BD 1 Frequency 2 (MHz)"() -> (w3474:dbl)
        n2215 = Multiply(x=w3484, y=w3483) -> (x*y=w3481:dbl)
        n2216 = Multiply(x=w3482, y=w3481) -> (x*y=w3480:dbl)
        n2217 = Scale By Power Of 2(n=-48, x=w3480) -> (x*2^n=w3478:dbl)
        n2218 = Divide(x=w3478, y=1000000.0) -> (x/y=w3475:dbl)
        n2219 = Subtract(x=w3474, y=w3475) -> (x-y=w3462:dbl)
        n2220 = local read "Target Force (pN)"() -> (w3473:dbl)
        n2221 = local read "T1 calibration"() -> (w3471:T12)
        n2222 = local read "Offset file step size"() -> (w3461:dbl)
        n2223 = local read "Setpoint offset\ncorrection values"() -> (w3458:dbl[])
        n2224 = Unbundle By Name(w3471) -> ("alpha_x (nm/V)"=w3470:dbl, "kappa_x (pN/nm)"=w3469:dbl)
        n2225 = Multiply(x=w3473, y=2.0) -> (x*y=w3467:dbl)
        n2226 = Divide(x=w3462, y=w3461) -> (x/y=w3460:dbl)
        n2227 = local read "Negate Diff?"() -> (w3464:bool)
        n2228 = To Long Integer(number=w3460) -> (32bit integer=w3459:i32)
        n2229 = Multiply(x=w3470, y=w3469) -> (x*y=w3468:dbl)
        n2230 = Index Array(array=w3458, index=w3459) -> (element=w3456:dbl)
        n2231 = Divide(x=w3467, y=w3468) -> (x/y=w3463:dbl)
        n2232 = Select(t=1, s=w3464, f=-1) -> (s? t:f=w3457:i32)
        n2233 = Multiply(x=w3457, y=w3456) -> (x*y=w3455:dbl)
        n2234 = Add(x=w3463, y=w3455) -> (x+y=w3454:dbl)
        n2235 = To Fixed-Point(number=w3454) -> (fixed-point=w3453:fxp<+/-,16,1>)  [unwired: 1 in]
        n2236 = property on="Trap Pos FB SP" class="DigNum (strict)"("Val(Sgnl)"=w3453) -> ()  [unwired: 2 in, 2 out]
      }
      event "Trap 3 (ON/OFF)", "T3 Y (V)", "T3 X (V)": Value Change {
        n2237 = event-data() -> ()  [unwired: 7 out]
        n2238 = Multiply(x="T3 X (V)", y=32767.0) -> (x*y=w3504:dbl)
        n2239 = Multiply(x="T3 Y (V)", y=32767.0) -> (x*y=w3501:dbl)
        n2240 = Divide(x=w3504, y=10.0) -> (x/y=w3505:dbl)
        n2241 = Divide(x=w3501, y=10.0) -> (x/y=w3500:dbl)
        n2242 = To Word Integer(number=w3505) -> (16bit integer=w3494:i16)
        n2243 = To Word Integer(number=w3500) -> (16bit integer=w3495:i16)
        n2244 = case shown="False" "Trap 3 (ON/OFF)" {
          tunnel: [5.0 0.0] -> w3488
          frame False {
          }
          frame True {
          }
        }
        n2245 = Multiply(x=w3488, y=32767.0) -> (x*y=w3491:dbl)
        n2246 = Divide(x=w3491, y=10.0) -> (x/y=w3490:dbl)
        n2247 = To Word Integer(number=w3490) -> (16bit integer=w3487:i16)
        n2248 = xnode "Read/Write Control"("FPGA VI Reference In"=w3496, "Piezo Trap X (AO5)"=w3494, "Piezo Trap Y (AO4)"=w3495, "Piezo Trap ON/Off (AO3)"=w3487) -> ()  [unwired: 1 in, 2 out]
      }
      event "Cursor control.X", "Cursor control.Y": Value Change {
        # "If turning cursor control off, update the piezo controls"
        n2249 = event-data() -> ()  [unwired: 7 out]
        n2250 = xnode "Read/Write Control"("FPGA VI Reference In"=w3515) -> ("Piezo X out"=w3513:i16, "Piezo Y out"=w3509:i16)  [unwired: 1 in, 2 out]
        n2251 = local read "Cursor control"() -> (w3514:cluster{"X":bool, "Y":bool})
        n2252 = Unbundle By Name(w3514) -> ("X"=w3512:bool, "Y"=w3511:bool)
        n2253 = And(x=w3512, y=w3511) -> (x .and. y?=w3510:bool)
        n2254 = case shown="True" w3510 {
          tunnel: w3513 -> [w3520 _]
          tunnel: w3509 -> [w3518 _]
          frame False {
            w3517 = 3276.7
            n2255 = Divide(x=w3520, y=w3517) -> (x/y=w3519:dbl)
            n2256 = Divide(x=w3518, y=w3517) -> (x/y=w3516:dbl)
            n2257 = property on="T3 X (V)" class="DigNum (strict)"("Val(Sgnl)"=w3519) -> ()  [unwired: 2 in, 2 out]
            n2258 = property on="T3 Y (V)" class="DigNum (strict)"("Val(Sgnl)"=w3516) -> ()  [unwired: 2 in, 2 out]
          }
          frame True {
          }
        }
      }
      event "MCL offset scanning range (V)": Value Change {
        n2259 = event-data() -> ()  [unwired: 7 out]
        n2260 = local read "Multiple-MCL offset?"() -> (w3521:bool)
        n2261 = case shown="False" w3521 {
          frame False {
            # "Initialize the multi-MCL offset array"
            n2262 = local read "MCL offset scanning range (V)"() -> (w3527:T4)
            n2263 = local read "Offset file step size"() -> (w3523:dbl)
            n2264 = Divide(x=30.0, y=w3523) -> (x/y=w3524:dbl)
            n2265 = Initialize Array(0.0, w3524) -> (w3526:dbl[])
            n2266 = call "Make Trap3 position array.vi"("MCL offset scanning range (V)"=w3527) -> ("X Data points"=w3530:u64, "Y data points"=w3532:u64)  [unwired: 3 out]
            n2267 = Bundle(w3526, w3526, w3526, w3526, w3526, w3526) -> (w3529:T50)  [unwired: 1 in]
            n2268 = Multiply(x=w3532, y=w3530) -> (x*y=w3528:u64)
            n2269 = for {
              N: w3528 -> [_]
              tunnel: [w3534] -> w3531 mode=indexing
              tunnel: w3529 -> [w3534]
            }
            n2270 = Reshape Array(w3531, w3530, w3532) -> (w3533:T51)
            n2271 = local write "Multi-MCL offset array"(w3533) -> ()
          }
          frame True {
            n2272 = flat-sequence {
              frame #0 {
                n2273 = property on="Multiple-MCL offset?" class="Bool (strict)"("Val(Sgnl)"=FALSE) -> ()  [unwired: 2 in, 2 out]
              }
              frame #1 {
                n2274 = Wait (ms)(milliseconds to wait=200) -> ()  [unwired: 1 out]
              }
              frame #2 {
                # "Initialize the multi-MCL offset array"
                n2275 = local read "MCL offset scanning range (V)"() -> (w3542:T4)
                n2276 = local read "Offset file step size"() -> (w3538:dbl)
                n2277 = Divide(x=30.0, y=w3538) -> (x/y=w3539:dbl)
                n2278 = Initialize Array(0.0, w3539) -> (w3541:dbl[])
                n2279 = call "Make Trap3 position array.vi"("MCL offset scanning range (V)"=w3542) -> ("X Data points"=w3545:u64, "Y data points"=w3547:u64)  [unwired: 3 out]
                n2280 = Bundle(w3541, w3541, w3541, w3541, w3541, w3541) -> (w3544:T50)  [unwired: 1 in]
                n2281 = Multiply(x=w3547, y=w3545) -> (x*y=w3543:u64)
                n2282 = for {
                  N: w3543 -> [_]
                  tunnel: [w3549] -> w3546 mode=indexing
                  tunnel: w3544 -> [w3549]
                }
                n2283 = Reshape Array(w3546, w3545, w3547) -> (w3548:T51)
                n2284 = local write "Multi-MCL offset array"(w3548) -> ()
              }
              frame #3 {
                n2285 = Wait (ms)(milliseconds to wait=200) -> ()  [unwired: 1 out]
              }
              frame #4 {
                n2286 = property on="Multiple-MCL offset?" class="Bool (strict)"("Val(Sgnl)"=TRUE) -> ()  [unwired: 2 in, 2 out]
              }
            }
          }
        }
      }
      event "2D force calibration": Value Change {
        n2287 = event-data() -> ()  [unwired: 7 out]
        n2288 = local read "2D force calibration"() -> (w3552:u16)
        n2289 = case shown="1" w3552 {
          tunnel: ["Position (V)" ("Label.Text") "Position (nm)" ("Label.Text") "Force (pN)" ("Label.Text")] -> w3553
          frame 0, Default {
          }
          frame 1 {
          }
          frame 2 {
          }
        }
        n2290 = property on="2D forces" class="WFChart (strict)"("YScale.NameLbl.Text"=w3553) -> ()  [unwired: 2 in, 2 out]
      }
      event "T3 positioning test range (V)": Value Change {
        n2291 = event-data() -> ()  [unwired: 7 out]
        n2292 = flat-sequence {
          frame #0 {
            n2293 = local read "T3 positioning test range (V)"() -> (w3559:T10)
            n2294 = control-ref of="Correlations in X"() -> (w3558:refnum<vi>)
            n2295 = control-ref of="Correlations in Y"() -> (w3557:refnum<vi>)
            n2296 = Unbundle By Name(w3559) -> ("Xmin"=w3567:dbl, "increment"=w3572:dbl, "Ymin"=w3568:dbl, "Xmax"=w3569:dbl, "Ymax"=w3571:dbl)
            n2297 = Unbundle By Name(w3559) -> ("Xmin"=w3560:dbl, "increment"=w3565:dbl, "Ymin"=w3563:dbl, "Xmax"=w3561:dbl, "Ymax"=w3564:dbl)
            n2298 = Add(x=w3572, y=w3569) -> (x+y=w3570:dbl)
            n2299 = Add(x=w3572, y=w3571) -> (x+y=w3573:dbl)
            n2300 = Add(x=w3561, y=w3565) -> (x+y=w3562:dbl)
            n2301 = Add(x=w3564, y=w3565) -> (x+y=w3566:dbl)
            n2302 = property on="Property Node" class="IntGraph (strict)"(reference=w3557, "XScale.Minimum"=w3567, "XScale.Maximum"=w3570, "YScale.Minimum"=w3568, "YScale.Maximum"=w3573) -> ()  [unwired: 1 in, 2 out]
            n2303 = property on="Property Node" class="IntGraph (strict)"(reference=w3558, "XScale.Minimum"=w3560, "XScale.Maximum"=w3562, "YScale.Minimum"=w3563, "YScale.Maximum"=w3566) -> ()  [unwired: 1 in, 2 out]
          }
          frame #1 {
            n2304 = Wait (ms)(milliseconds to wait=50) -> ()  [unwired: 1 out]
          }
          frame #2 {
            n2305 = local read "T3 positioning test range (V)"() -> (w3577:T10)
            n2306 = control-ref of="Correlations in X"() -> (w3576:refnum<vi>)
            n2307 = control-ref of="Correlations in Y"() -> (w3575:refnum<vi>)
            n2308 = Unbundle By Name(w3577) -> ("Xmin"=w3581:dbl, "increment"=w3583:dbl, "Ymin"=w3582:dbl)
            n2309 = Unbundle By Name(w3577) -> ("Xmin"=w3578:dbl, "increment"=w3580:dbl, "Ymin"=w3579:dbl)
            n2310 = property on="Property Node" class="IntGraph (strict)"(reference=w3575, "XScale.Offset"=w3581, "XScale.Multiplier"=w3583, "YScale.Offset"=w3582, "YScale.Multiplier"=w3583) -> ()  [unwired: 1 in, 2 out]
            n2311 = property on="Property Node" class="IntGraph (strict)"(reference=w3576, "XScale.Offset"=w3578, "XScale.Multiplier"=w3580, "YScale.Offset"=w3579, "YScale.Multiplier"=w3580) -> ()  [unwired: 1 in, 2 out]
          }
        }
      }
      event "Scale intensities": Value Change {
        n2312 = event-data() -> ()  [unwired: 7 out]
        n2313 = local read "T2 calibration"() -> (w3591:T12)
        n2314 = local read "T1 calibration"() -> (w3584:T12)